vi "SMain.vi"() -> ()   [LabVIEW 2011] (continued)
0.283628\t0.245762\t0.211217\t0.212405\t0.226173\t0.234537\t0.236943\t0.231864\t0.218697\t0.203239\t0.212648\t0.219975\t0.225754\t0.228965\t0.229842\t0.227372\t0.235008\t0.246799\t0.255143\t0.261054\t0.264959\t0.267617\t0.269243\t0.269330\t0.267908\t0.264189\t0.257117\t0.251459\t0.263708\t0.269155\t0.266275\t0.292834\t0.323832\t0.346673\t0.359823\t0.362859\t0.356143\t0.340301\t0.316382\t0.287617\t0.273147\t0.255370\t0.232779\t0.205366\t0.184259\t0.170019\t0.153921\t0.138670\t0.147883\t0.157027\t0.165968\t0.178336\t0.204158\t0.226001\t0.243359\t0.256761\t0.265807\t0.270629\t0.271087\t0.271595\t0.274347\t0.273205\t0.284365\t0.290284\t0.291349\t0.282591\t0.268256\t0.253620\t0.246165\t0.249064\t0.246551\t0.238815\t0.226554\t0.210821\t0.192072\t0.170652\t0.155599\t0.155342\t0.161398\t0.165827\t0.167815\t0.166899\t0.173033\t0.183751\t0.192188\t0.212259\t0.241683\t0.269258\t0.293587\t0.314870\t0.333907\t0.351562\t0.368177\t0.383535\t0.397109\t0.407462\t0.412280\t0.409681\t0.419271\t0.438212\t0.456536\t0.460520\t0.453373\t0.437822\t0.419330\t0.400059\t0.375598\t0.345922\t0.315517\t0.294393\t0.276275\t0.256682\t0.235989\t0.212984\t0.221098\t0.231416\t0.236020\t0.246406\t0.268197\t0.283488\t0.291798\t0.294021\t0.290269\t0.280164\t0.264732\t0.299218\t0.335759\t0.373895\t0.412717\t0.447558\t0.468282\t0.461593\t0.427812\t0.447950\t0.482415\t0.501348\t0.510509\t0.512644\t0.508751\t0.498815\t0.483536\t0.485993\t0.477612\t0.457996\t0.425809\t0.384493\t0.344197\t0.326015\t0.302418\t0.272693\t0.237314\t0.216368\t0.210999\t0.199478\t0.207422\t0.232209\t0.251430\t0.266692\t0.284547\t0.301564\t0.329963\t0.366754\t0.402163\t0.427979\t0.426160\t0.475391\t0.545419\t0.537304\t0.479878\t0.459344\t0.451837\t0.454875\t0.465103\t0.478472\t0.489788\t0.494041\t0.487578\t0.468860\t0.438519\t0.399262\t0.353683\t0.305159\t0.285243\t0.282794\t0.274771\t0.260306\t0.239832\t0.212870\t0.186954\t0.181018\t0.172682\t0.162741\t0.164205\t0.181691\t0.197406\t0.217042\t0.241977\t0.265612\t0.291513\t0.357547\t0.416207\t0.466336\t0.534557\t0.484360\t0.426967\t0.399242\t0.390179\t0.380132\t0.376954\t0.366830\t0.349703\t0.326406\t0.298792\t0.270192\t0.250152\t0.237509\t0.223353\t0.207727\t0.191599\t0.198789\t0.207616\t0.242361\t0.266834\t0.281833\t0.287549\t0.284975\t0.274905\t0.258380\t0.235371\t0.206881\t0.203974\t0.229886\t0.255407\t0.280368\t0.310090\t0.346393\t0.328419\t0.547614\t0.529029\t0.416521\t0.384530\t0.347957\t0.317457\t0.289868\t0.261307\t0.245565\t0.261859\t0.294259\t0.327642\t0.358488\t0.365440\t0.348072\t0.309690\t0.255227\t0.240856\t0.244745\t0.245644\t0.243448\t0.267308\t0.282974\t0.288154\t0.284990\t0.275718\t0.261981\t0.265585\t0.277745\t0.291323\t0.306635\t0.334255\t0.362487\t0.382155\t0.353107\t0.253723\t0.328487\t0.577657\t0.533197\t0.444535\t0.396380\t0.364336\t0.339954\t0.349876\t0.362823\t0.384932\t0.406211\t0.413308\t0.403604\t0.377026\t0.337623\t0.289783\t0.272802\t0.257998\t0.243067\t0.227691\t0.221062\t0.216984\t0.213519\t0.223928\t0.234176\t0.242151\t0.248691\t0.253760\t0.258533\t0.263086\t0.267987\t0.273321\t0.287187\t0.311427\t0.320659\t0.286503\t0.237761\t0.343422\t0.397936\t0.389088\t0.372420\t0.361320\t0.354887\t0.367300\t0.377100\t0.380880\t0.381876\t0.383263\t0.385396\t0.387321\t0.387314\t0.384670\t0.378768\t0.373171\t0.363294\t0.348426\t0.328810\t0.313661\t0.308140\t0.297820\t0.282779\t0.263614\t0.241021\t0.215664\t0.214650\t0.218524\t0.229368\t0.253303\t0.273400\t0.292726\t0.295180\t0.280740\t0.235075\t0.247165\t0.271864\t0.272601\t0.263658\t0.258491\t0.263036\t0.264623\t0.267156\t0.272119\t0.286296\t0.307948\t0.326343\t0.339551\t0.347695\t0.356165\t0.365090\t0.365929\t0.359185\t0.345101\t0.324021\t0.297159\t0.290971\t0.280471\t0.265929\t0.248134\t0.226787\t0.219501\t0.263268\t0.311418\t0.359460\t0.406412\t0.446072\t0.458457\t0.418051\t0.344402\t0.280814\t0.230547\t0.208763\t0.198393\t0.193984\t0.208428\t0.213708\t0.210549\t0.232831\t0.253343\t0.270174\t0.282384\t0.288428\t0.289253\t0.284449\t0.278158\t0.286162\t0.291709\t0.290978\t0.284685\t0.271977\t0.261930\t0.261843\t0.260557\t0.272878\t0.283097\t0.291201\t0.297702\t0.324738\t0.371822\t0.417347\t0.457160\t0.481983\t0.480434\t0.450945\t0.404940\t0.353302\t0.301366\t0.250340\t0.199463\t0.149905\t0.148044\t0.164917\t0.193805\t0.216060\t0.231730\t0.241425\t0.245345\t0.251396\t0.261354\t0.272109\t0.277008\t0.273982\t0.263905\t0.248095\t0.229016\t0.209334\t0.206918\t0.200256\t0.189194\t0.178563\t0.201006\t0.223512\t0.256966\t0.308178\t0.367285\t0.414461\t0.444076\t0.452547\t0.440556\t0.413079\t0.375352\t0.330473\t0.279915\t0.224559\t0.238179\t0.268251\t0.289701\t0.303694\t0.311106\t0.323498\t0.342296\t0.355783\t0.363059\t0.364734\t0.372386\t0.382440\t0.387105\t0.386380\t0.380014\t0.367984\t0.354404\t0.334320\t0.305024\t0.270724\t0.253479\t0.229524\t0.240661\t0.278172\t0.303423\t0.309321\t0.327805\t0.352880\t0.365338\t0.363062\t0.345545\t0.341657\t0.327248\t0.302778\t0.298982\t0.305407\t0.328732\t0.351562\t0.367323\t0.377527\t0.381915\t0.380700\t0.389886\t0.411792\t0.429718\t0.443070\t0.452189\t0.462028\t0.484533\t0.500970\t0.511585\t0.516472\t0.514869\t0.506859\t0.490042\t0.463092\t0.423348\t0.387697\t0.420283\t0.472795\t0.503287\t0.496605\t0.466110\t0.425165\t0.380234\t0.405919\t0.428246\t0.440520\t0.443040\t0.436016\t0.445391\t0.459226\t0.464376\t0.461519\t0.463782\t0.470042\t0.477734\t0.478099\t0.471522\t0.457734\t0.436599\t0.407482\t0.409522\t0.412435\t0.410855\t0.409858\t0.441504\t0.471085\t0.494884\t0.511916\t0.520217\t0.515811\t0.493593\t0.461473\t0.504275\t0.528907\t0.545940\t0.525848\t0.492871\t0.457356\t0.421811\t0.390188\t0.421623\t0.444622\t0.459503\t0.466499\t0.465399\t0.485211\t0.508342\t0.522057\t0.529166\t0.532661\t0.528202\t0.516283\t0.497511\t0.477618\t0.455396\t0.429103\t0.409839\t0.422814\t0.433580\t0.441468\t0.445063\t0.441505\t0.425413\t0.423568\t0.444595\t0.469483\t0.470244\t0.504422\t0.538810\t0.510307\t0.481224\t0.464360\t0.435482\t0.401512\t0.365738\t0.351663\t0.347792\t0.374340\t0.394838\t0.410657\t0.422636\t0.428568\t0.455461\t0.473935\t0.486501\t0.489080\t0.483415\t0.472741\t0.455953\t0.435971\t0.414313\t0.388283\t0.356923\t0.319829\t0.303499\t0.304199\t0.299926\t0.317529\t0.357519\t0.387193\t0.400232\t0.416388\t0.500520\t0.560550\t0.540864\t0.459527\t0.362457\t0.272386\t0.273714\t0.283399\t0.288175\t0.289507\t0.287334\t0.329713\t0.382820\t0.427099\t0.462841\t0.490597\t0.510557\t0.523304\t0.529592\t0.529644\t0.524214\t0.513381\t0.497513\t0.476542\t0.450552\t0.419506\t0.383069\t0.340788\t0.314518\t0.301862\t0.285418\t0.263462\t0.286474\t0.325141\t0.370395\t0.457672\t0.528673\t0.581745\t0.630440\t0.558222\t0.459605\t0.359034\t0.256043\t0.186353\t0.196527\t0.223114\t0.287556\t0.343482\t0.392027\t0.433151\t0.466912\t0.493138\t0.511885\t0.522375\t0.525247\t0.522661\t0.516170\t0.503255\t0.483593\t0.457521\t0.424744\t0.385247\t0.337875\t0.281986\t0.222332\t0.196464\t0.168315\t0.199827\t0.297894\t0.393688\t0.485674\t0.566418\t0.602390\t0.561914\t0.536383\t0.468234\t0.383735\t0.290171\t0.203294\t0.178384\t0.210509\t0.252834\t0.291136\t0.351988\t0.406299\t0.454014\t0.493145\t0.522706\t0.543349\t0.556171\t0.560777\t0.558044\t0.548310\t0.531609\t0.507914\t0.477059\t0.438688\t0.391758\t0.335510\t0.268462\t0.189937\t0.194836\t0.216142\t0.289303\t0.380077\t0.463169\t0.533036\t0.576586\t0.575110\t0.565734\t0.519516\t0.453580\t0.377901\t0.295142\t0.217327\t0.224530\t0.241548\t0.258810\t0.298433\t0.340211\t0.392148\t0.436929\t0.471555\t0.496820\t0.513586\t0.521902\t0.522678\t0.516093\t0.501947\t0.480688\t0.452230\t0.415769\t0.370593\t0.315865\t0.250062\t0.208029\t0.202220\t0.273491\t0.343790\t0.412406\t0.478453\t0.523029\t0.531626\t0.504386\t0.469927\t0.427337\t0.366285\t0.293579\t0.246633\t0.199839\t0.193240\t0.229121\t0.278636\t0.321381\t0.363778\t0.397804\t0.424215\t0.451528\t0.473408\t0.486991\t0.492257\t0.489773\t0.479697\t0.462200\t0.436921\t0.403425\t0.360622\t0.307463\t0.243094\t0.184691\t0.209702\t0.251723\t0.325476\t0.400921\t0.470003\t0.530259\t0.571112\t0.573487\t0.534825\t0.475632\t0.409566\t0.336649\t0.257237\t0.197933\t0.209001\t0.214909\t0.216695\t0.256190\t0.324325\t0.381754\t0.429322\t0.467371\t0.495988\t0.515274\t0.525368\t0.526234\t0.520614\t0.508597\t0.488112\t0.458790\t0.419525\t0.369464\t0.307098\t0.238203\t0.242228\t0.265368\t0.300661\t0.344032\t0.410603\t0.479673\t0.534824\t0.571454\t0.602830\t0.596127\t0.555797\t0.497616\t0.429305\t0.369440\t0.362815\t0.348104\t0.334447\t0.344405\t0.359822\t0.388094\t0.413667\t0.433616\t0.447982\t0.477571\t0.510696\t0.535494\t0.556379\t0.568836\t0.572953\t0.567774\t0.552167\t0.524242\t0.482388\t0.424709\t0.349650\t0.281009\t0.293141\t0.324182\t0.376542\t0.428911\t0.469606\t0.504124\t0.525933\t0.566340\t0.582894\t0.565709\t0.526939\t0.476831\t0.419808\t0.356430\t0.375996\t0.389325\t0.394846\t0.438324\t0.471657\t0.494369\t0.508208\t0.514595\t0.514534\t0.508563\t0.503983\t0.493846\t0.476518\t0.482266\t0.493088\t0.498311\t0.498172\t0.491813\t0.477354\t0.450623\t0.419694\t0.420469\t0.406702\t0.449165\t0.484928\t0.537284\t0.568439\t0.564549\t0.526264\t0.513586\t0.483592\t0.436907\t0.408022\t0.371531\t0.330444\t0.285175\t0.269758\t0.314643\t0.382234\t0.437532\t0.481159\t0.513885\t0.536591\t0.549875\t0.554426\t0.550873\t0.539049\t0.519095\t0.490678\t0.452702\t0.404557\t0.345193\t0.279027\t0.208926\t0.188780\t0.204172\t0.285686\t0.356868\t0.417221\t0.464399\t0.495873\t0.549856\t0.578829\t0.568718\t0.527730\t0.470061\t0.402511\t0.344606\t0.281995\t0.231645\t0.219810\t0.208184\t0.213811\t0.261394\t0.306970\t0.358330\t0.405302\t0.442232\t0.469227\t0.487278\t0.496263\t0.496249\t0.487766\t0.470779\t0.445359\t0.411061\t0.367520\t0.351049\t0.349671\t0.370138\t0.381358\t0.418282\t0.450278\t0.473128\t0.483470\t0.478606\t0.475260\t0.479347\t0.483894\t0.466262\t0.439077\t0.399049\t0.350279\t0.356069\t0.385474\t0.407836\t0.429011\t0.450986\t0.462125\t0.477665\t0.489562\t0.492232\t0.487732\t0.476318\t0.458745\t0.451629\t0.447323\t0.433005\t0.408337\t0.372742\t0.326121\t0.302166\t0.275420\t0.283692\t0.335462\t0.375904\t0.405174\t0.444641\t0.477024\t0.509659\t0.527287\t0.528099\t0.512153\t0.480891\t0.446450\t0.405819\t0.370155\t0.325004\t0.317091\t0.329503\t0.333984\t0.352630\t0.380560\t0.396845\t0.402644\t0.452431\t0.496921\t0.531289\t0.555002\t0.566928\t0.565978\t0.551443\t0.522857\t0.480125\t0.432074\t0.412920\t0.388243\t0.366711\t0.391066\t0.441269\t0.496425\t0.545376\t0.582830\t0.604194\t0.643929\t0.648619\t0.615624\t0.573572\t0.524660\t0.470410\t0.409949\t0.341730\t0.333469\t0.320281\t0.338808\t0.377347\t0.450598\t0.521221\t0.577536\t0.612709\t0.620570\t0.607012\t0.585988\t0.569740\t0.596697\t0.615589\t0.625074\t0.624250\t0.611104\t0.583775\t0.541273\t0.482818\t0.425523\t0.402684\t0.375029\t0.405172\t0.472541\t0.534364\t0.589427\t0.631385\t0.644305\t0.696630\t0.726898\t0.670819\t0.611493\t0.553228\t0.496096\t0.435503\t0.369117\t0.326541\t0.322722\t0.365619\t0.455135\t0.537005\t0.604795\t0.650551\t0.659845\t0.634266\t0.589969\t0.544563\t0.543038\t0.566033\t0.579752\t0.583902\t0.577357\t0.559192\t0.528044\t0.482959\t0.473916\t0.467569\t0.466798\t0.516529\t0.565986\t0.625401\t0.682654\t0.738689\t0.768686\t0.723737\t0.664643\t0.668513\t0.648942\t0.606669\t0.548689\t0.478729\t0.416653\t0.393396\t0.405301\t0.463639\t0.502262\t0.521920\t0.541442\t0.615764\t0.679112\t0.717213\t0.697073\t0.643352\t0.580514\t0.538723\t0.543622\t0.542648\t0.534707\t0.528432\t0.530172\t0.518495\t0.496118\t0.464957\t0.480032\t0.524973\t0.563766\t0.586576\t0.591948\t0.596186\t0.626183\t0.644569\t0.644771\t0.622742\t0.582121\t0.547187\t0.503721\t0.452912\t0.395361\t0.399924\t0.416756\t0.427056\t0.462622\t0.483459\t0.485498\t0.521835\t0.571251\t0.601303\t0.599222\t0.563134\t0.504997\t0.456226\t0.472383\t0.494940\t0.539548\t0.568317\t0.572056\t0.553244\t0.519514\t0.476010\t0.453420\t0.489455\t0.519267\t0.531145\t0.525721\t0.505641\t0.474430\t0.460246\t0.438145\t0.428223\t0.421217\t0.407486\t0.388276\t0.386569\t0.410844\t0.429081\t0.440012\t0.441823\t0.432587\t0.414508\t0.407526\t0.437521\t0.473799\t0.498390\t0.506650\t0.494787\t0.461595\t0.409666\t0.341647\t0.373382\t0.442667\t0.508897\t0.575264\t0.642191\t0.663048\t0.598512\t0.521720\t0.441507\t0.397262\t0.401391\t0.396607\t0.383886\t0.364256\t0.361834\t0.382014\t0.393293\t0.396638\t0.408296\t0.435949\t0.453622\t0.461256\t0.458790\t0.446197\t0.423763\t0.391947\t0.351378\t0.325228\t0.323591\t0.332213\t0.331860\t0.321746\t0.300427\t0.279036\t0.285285\t0.289284\t0.348673\t0.402814\t0.454151\t0.505876\t0.560490\t0.619477\t0.648206\t0.581997\t0.490788\t0.392154\t0.327889\t0.294591\t0.241517\t0.183914\t0.244860\t0.340821\t0.417223\t0.476339\t0.519139\t0.545132\t0.553091\t0.543649\t0.520182\t0.486447\t0.445854\t0.400016\t0.348705\t0.317378\t0.296637\t0.270253\t0.253022\t0.256487\t0.281300\t0.329629\t0.373549\t0.405454\t0.423140\t0.426175\t0.467618\t0.500448\t0.524604\t0.578041\t0.648927\t0.768815\t0.611204\t0.499742\t0.385965\t0.410939\t0.460363\t0.476248\t0.427084\t0.382432\t0.431486\t0.510854\t0.571616\t0.609242\t0.616236\t0.597115\t0.564786\t0.526904\t0.485527\t0.441142\t0.393066\t0.340714\t0.312720\t0.283130\t0.274617\t0.317943\t0.365852\t0.415609\t0.463028\t0.501034\t0.520392\t0.514781\t0.487333\t0.470956\t0.477926\t0.469899\t0.455372\t0.496003\t0.556269\t0.638059\t0.657762\t0.523704\t0.437292\t0.379563\t0.477568\t0.547877\t0.547803\t0.554779\t0.608169\t0.629652\t0.608660\t0.569138\t0.530166\t0.495117\t0.458057\t0.418250\t0.374444\t0.326581\t0.304486\t0.309894\t0.325427\t0.338649\t0.352519\t0.382272\t0.437265\t0.511846\t0.575378\t0.602752\t0.576762\t0.527943\t0.476567\t0.426531\t0.377757\t0.402903\t0.426040\t0.446072\t0.460736\t0.464301\t0.459479\t0.466591\t0.455818\t0.520123\t0.576969\t0.642519\t0.698880\t0.708516\t0.671105\t0.628935\t0.586976\t0.543354\t0.496169\t0.443443\t0.383189\t0.337040\t0.340225\t0.342015\t0.383194\t0.434352\t0.481352\t0.516829\t0.541320\t0.535486\t0.534695\t0.603454\t0.636773\t0.614150\t0.567494\t0.517425\t0.467899\t0.440850\t0.440765\t0.432974\t0.415287\t0.400566\t0.410859\t0.468748\t0.527456\t0.583222\t0.623550\t0.654776\t0.664060\t0.647281\t0.612904\t0.568995\t0.522635\t0.481019\t0.433459\t0.378471\t0.315361\t0.243094\t0.248332\t0.307193\t0.377542\t0.451180\t0.530402\t0.620129\t0.720620\t0.647989\t0.563797\t0.513044\t0.540331\t0.547544\t0.534369\t0.506213\t0.468360\t0.472190\t0.474080\t0.467050\t0.459976\t0.471495\t0.506108\t0.561024\t0.608718\t0.643715\t0.656606\t0.643965\t0.615051\t0.577670\t0.534509\r\n*0.000000\t0.001250\t0.002501\t0.003751\t0.005001\t0.006252\t0.007502\t0.008752\t0.010003\t0.011253\t0.012503\t0.013753\t0.015004\t0.016254\t0.017504\t0.018755\t0.020005\t0.021255\t0.022506\t0.023756\t0.025006\t0.026257\t0.027507\t0.028757\t0.030008\t0.031258\t0.032508\t0.033758\t0.035009\t0.036259\t0.037509\t0.038760\t0.040010\t0.041260\t0.042511\t0.043761\t0.045011\t0.046262\t0.047512\t0.048762\t0.050013\t0.051263\t0.052513\t0.053763\t0.055014\t0.056264\t0.057514\t0.058765\t0.060015\t0.061265\t0.062516\t0.063766\t0.065016\t0.066267\t0.067517\t0.068767\t0.070018\t0.071268\t0.072518\t0.073768\t0.075019\t0.076269\t0.077519\t0.078770\t0.080020\t0.081270\t0.082521\t0.083771\t0.085021\t0.086272\t0.087522\t0.088772\t0.090023\t0.091273\t0.092523\t0.093773\t0.095024\t0.096274\t0.097524\t0.098775\t0.100025\t0.101275\t0.102526\t0.103776\t0.105026\t0.106277\t0.107527\t0.108777\t0.110028\t0.111278\t0.112528\t0.113778\t0.115029\t0.116279\t0.117529\t0.118780\t0.120030\t0.121280\t0.122531\t0.123781\t0.125031\t0.126282\t0.127532\t0.128782\t0.130033\t0.131283\t0.132533\t0.133783\t0.135034\t0.136284\t0.137534\t0.138785\t0.140035\t0.141285\t0.142536\t0.143786\t0.145036\t0.146287\t0.147537\t0.148787\t0.150038\t0.151288\t0.152538\t0.153788\t0.155039\t0.156289\t0.157539\t0.158790\t0.160040\t0.161290\t0.162541\t0.163791\t0.165041\t0.166292\t0.167542\t0.168792\t0.170043\t0.171293\t0.172543\t0.173793\t0.175044\t0.176294\t0.177544\t0.178795\t0.180045\t0.181295\t0.182546\t0.183796\t0.185046\t0.186297\t0.187547\t0.188797\t0.190048\t0.191298\t0.192548\t0.193798\t0.195049\t0.196299\t0.197549\t0.198800\t0.200050\t0.201300\t0.202551\t0.203801\t0.205051\t0.206302\t0.207552\t0.208802\t0.210053\t0.211303\t0.212553\t0.213803\t0.215054\t0.216304\t0.217554\t0.218805\t0.220055\t0.221305\t0.222556\t0.223806\t0.225056\t0.226307\t0.227557\t0.228807\t0.230058\t0.231308\t0.232558\t0.233808\t0.235059\t0.236309\t0.237559\t0.238810\t0.240060\t0.241310\t0.242561\t0.243811\t0.245061\t0.246312\t0.247562\t0.248812\t0.250063\t0.251313\t0.252563\t0.253813\t0.255064\t0.256314\t0.257564\t0.258815\t0.260065\t0.261315\t0.262566\t0.263816\t0.265066\t0.266317\t0.267567\t0.268817\t0.270068\t0.271318\t0.272568\t0.273818\t0.275069\t0.276319\t0.277569\t0.278820\t0.280070\t0.281320\t0.282571\t0.283821\t0.285071\t0.286322\t0.287572\t0.288822\t0.290073\t0.291323\t0.292573\t0.293823\t0.295074\t0.296324\t0.297574\t0.298825\t0.300075\t0.301325\t0.302576\t0.303826\t0.305076\t0.306327\t0.307577\t0.308827\t0.310078\t0.311328\t0.312578\t0.313828\t0.315079\t0.316329\t0.317579\t0.318830\t0.320080\t0.321330\t0.322581\t0.323831\t0.325081\t0.326332\t0.327582\t0.328832\t0.330083\t0.331333\t0.332583\t0.333833\t0.335084\t0.336334\t0.337584\t0.338835\t0.340085\t0.341335\t0.342586\t0.343836\t0.345086\t0.346337\t0.347587\t0.348837\t0.350088\t0.351338\t0.352588\t0.353838\t0.355089\t0.356339\t0.357589\t0.358840\t0.360090\t0.361340\t0.362591\t0.363841\t0.365091\t0.366342\t0.367592\t0.368842\t0.370093\t0.371343\t0.372593\t0.373843\t0.375094\t0.376344\t0.377594\t0.378845\t0.380095\t0.381345\t0.382596\t0.383846\t0.385096\t0.386347\t0.387597\t0.388847\t0.390098\t0.391348\t0.392598\t0.393848\t0.395099\t0.396349\t0.397599\t0.398850\t0.400100\t0.401350\t0.402601\t0.403851\t0.405101\t0.406352\t0.407602\t0.408852\t0.410103\t0.411353\t0.412603\t0.413853\t0.415104\t0.416354\t0.417604\t0.418855\t0.420105\t0.421355\t0.422606\t0.423856\t0.425106\t0.426357\t0.427607\t0.428857\t0.430108\t0.431358\t0.432608\t0.433858\t0.435109\t0.436359\t0.437609\t0.438860\t0.440110\t0.441360\t0.442611\t0.443861\t0.445111\t0.446362\t0.447612\t0.448862\t0.450113\t0.451363\t0.452613\t0.453863\t0.455114\t0.456364\t0.457614\t0.458865\t0.460115\t0.461365\t0.462616\t0.463866\t0.465116\t0.466367\t0.467617\t0.468867\t0.470118\t0.471368\t0.472618\t0.473868\t0.475119\t0.476369\t0.477619\t0.478870\t0.480120\t0.481370\t0.482621\t0.483871\t0.485121\t0.486372\t0.487622\t0.488872\t0.490123\t0.491373\t0.492623\t0.493873\t0.495124\t0.496374\t0.497624\t0.498875\t0.500125\t0.501375\t0.502626\t0.503876\t0.505126\t0.506377\t0.507627\t0.508877\t0.510128\t0.511378\t0.512628\t0.513878\t0.515129\t0.516379\t0.517629\t0.518880\t0.520130\t0.521380\t0.522631\t0.523881\t0.525131\t0.526382\t0.527632\t0.528882\t0.530133\t0.531383\t0.532633\t0.533883\t0.535134\t0.536384\t0.537634\t0.538885\t0.540135\t0.541385\t0.542636\t0.543886\t0.545136\t0.546387\t0.547637\t0.548887\t0.550138\t0.551388\t0.552638\t0.553888\t0.555139\t0.556389\t0.557639\t0.558890\t0.560140\t0.561390\t0.562641\t0.563891\t0.565141\t0.566392\t0.567642\t0.568892\t0.570143\t0.571393\t0.572643\t0.573893\t0.575144\t0.576394\t0.577644\t0.578895\t0.580145\t0.581395\t0.582646\t0.583896\t0.585146\t0.586397\t0.587647\t0.588897\t0.590148\t0.591398\t0.592648\t0.593898\t0.595149\t0.596399\t0.597649\t0.598900\t0.600150\t0.601400\t0.602651\t0.603901\t0.605151\t0.606402\t0.607652\t0.608902\t0.610153\t0.611403\t0.612653\t0.613903\t0.615154\t0.616404\t0.617654\t0.618905\t0.620155\t0.621405\t0.622656\t0.623906\t0.625156\t0.626407\t0.627657\t0.628907\t0.630158\t0.631408\t0.632658\t0.633908\t0.635159\t0.636409\t0.637659\t0.638910\t0.640160\t0.641410\t0.642661\t0.643911\t0.645161\t0.646412\t0.647662\t0.648912\t0.650163\t0.651413\t0.652663\t0.653913\t0.655164\t0.656414\t0.657664\t0.658915\t0.660165\t0.661415\t0.662666\t0.663916\t0.665166\t0.666417\t0.667667\t0.668917\t0.670168\t0.671418\t0.672668\t0.673918\t0.675169\t0.676419\t0.677669\t0.678920\t0.680170\t0.681420\t0.682671\t0.683921\t0.685171\t0.686422\t0.687672\t0.688922\t0.690173\t0.691423\t0.692673\t0.693923\t0.695174\t0.696424\t0.697674\t0.698925\t0.700175\t0.701425\t0.702676\t0.703926\t0.705176\t0.706427\t0.707677\t0.708927\t0.710178\t0.711428\t0.712678\t0.713928\t0.715179\t0.716429\t0.717679\t0.718930\t0.720180\t0.721430\t0.722681\t0.723931\t0.725181\t0.726432\t0.727682\t0.728932\t0.730183\t0.731433\t0.732683\t0.733933\t0.735184\t0.736434\t0.737684\t0.738935\t0.740185\t0.741435\t0.742686\t0.743936\t0.745186\t0.746437\t0.747687\t0.748937\t0.750188\t0.751438\t0.752688\t0.753938\t0.755189\t0.756439\t0.757689\t0.758940\t0.760190\t0.761440\t0.762691\t0.763941\t0.765191\t0.766442\t0.767692\t0.768942\t0.770193\t0.771443\t0.772693\t0.773943\t0.775194\t0.776444\t0.777694\t0.778945\t0.780195\t0.781445\t0.782696\t0.783946\t0.785196\t0.786447\t0.787697\t0.788947\t0.790198\t0.791448\t0.792698\t0.793948\t0.795199\t0.796449\t0.797699\t0.798950\t0.800200\t0.801450\t0.802701\t0.803951\t0.805201\t0.806452\t0.807702\t0.808952\t0.810203\t0.811453\t0.812703\t0.813953\t0.815204\t0.816454\t0.817704\t0.818955\t0.820205\t0.821455\t0.822706\t0.823956\t0.825206\t0.826457\t0.827707\t0.828957\t0.830208\t0.831458\t0.832708\t0.833958\t0.835209\t0.836459\t0.837709\t0.838960\t0.840210\t0.841460\t0.842711\t0.843961\t0.845211\t0.846462\t0.847712\t0.848962\t0.850213\t0.851463\t0.852713\t0.853963\t0.855214\t0.856464\t0.857714\t0.858965\t0.860215\t0.861465\t0.862716\t0.863966\t0.865216\t0.866467\t0.867717\t0.868967\t0.870218\t0.871468\t0.872718\t0.873968\t0.875219\t0.876469\t0.877719\t0.878970\t0.880220\t0.881470\t0.882721\t0.883971\t0.885221\t0.886472\t0.887722\t0.888972\t0.890223\t0.891473\t0.892723\t0.893973\t0.895224\t0.896474\t0.897724\t0.898975\t0.900225\t0.901475\t0.902726\t0.903976\t0.905226\t0.906477\t0.907727\t0.908977\t0.910228\t0.911478\t0.912728\t0.913978\t0.915229\t0.916479\t0.917729\t0.918980\t0.920230\t0.921480\t0.922731\t0.923981\t0.925231\t0.926482\t0.927732\t0.928982\t0.930233\t0.931483\t0.932733\t0.933983\t0.935234\t0.936484\t0.937734\t0.938985\t0.940235\t0.941485\t0.942736\t0.943986\t0.945236\t0.946487\t0.947737\t0.948987\t0.950238\t0.951488\t0.952738\t0.953988\t0.955239\t0.956489\t0.957739\t0.958990\t0.960240\t0.961490\t0.962741\t0.963991\t0.965241\t0.966492\t0.967742\t0.968992\t0.970243\t0.971493\t0.972743\t0.973993\t0.975244\t0.976494\t0.977744\t0.978995\t0.980245\t0.981495\t0.982746\t0.983996\t0.985246\t0.986497\t0.987747\t0.988997\t0.990248\t0.991498\t0.992748\t0.993998\t0.995249\t0.996499\t0.997749\t0.999000\t1.000250\t1.001500\t1.002751\t1.004001\t1.005251\t1.006502\t1.007752\t1.009002\t1.010253\t1.011503\t1.012753\t1.014004\t1.015254\t1.016504\t1.017754\t1.019005\t1.020255\t1.021505\t1.022756\t1.024006\t1.025256\t1.026507\t1.027757\t1.029007\t1.030258\t1.031508\t1.032758\t1.034009\t1.035259\t1.036509\t1.037759\t1.039010\t1.040260\t1.041510\t1.042761\t1.044011\t1.045261\t1.046512\t1.047762\t1.049012\t1.050263\t1.051513\t1.052763\t1.054014\t1.055264\t1.056514\t1.057764\t1.059015\t1.060265\t1.061515\t1.062766\t1.064016\t1.065266\t1.066517\t1.067767\t1.069017\t1.070268\t1.071518\t1.072768\t1.074019\t1.075269\t1.076519\t1.077769\t1.079020\t1.080270\t1.081520\t1.082771\t1.084021\t1.085271\t1.086522\t1.087772\t1.089022\t1.090273\t1.091523\t1.092773\t1.094024\t1.095274\t1.096524\t1.097774\t1.099025\t1.100275\t1.101525\t1.102776\t1.104026\t1.105276\t1.106527\t1.107777\t1.109027\t1.110278\t1.111528\t1.112778\t1.114029\t1.115279\t1.116529\t1.117779\t1.119030\t1.120280\t1.121530\t1.122781\t1.124031\t1.125281\t1.126532\t1.127782\t1.129032\t1.130283\t1.131533\t1.132783\t1.134034\t1.135284\t1.136534\t1.137784\t1.139035\t1.140285\t1.141535\t1.142786\t1.144036\t1.145286\t1.146537\t1.147787\t1.149037\t1.150288\t1.151538\t1.152788\t1.154039\t1.155289\t1.156539\t1.157789\t1.159040\t1.160290\t1.161540\t1.162791\t1.164041\t1.165291\t1.166542\t1.167792\t1.169042\t1.170293\t1.171543\t1.172793\t1.174044\t1.175294\t1.176544\t1.177794\t1.179045\t1.180295\t1.181545\t1.182796\t1.184046\t1.185296\t1.186547\t1.187797\t1.189047\t1.190298\t1.191548\t1.192798\t1.194049\t1.195299\t1.196549\t1.197799\t1.199050\t1.200300\t1.201550\t1.202801\t1.204051\t1.205301\t1.206552\t1.207802\t1.209052\t1.210303\t1.211553\t1.212803\t1.214054\t1.215304\t1.216554\t1.217804\t1.219055\t1.220305\t1.221555\t1.222806\t1.224056\t1.225306\t1.226557\t1.227807\t1.229057\t1.230308\t1.231558\t1.232808\t1.234059\t1.235309\t1.236559\t1.237809\t1.239060\t1.240310\t1.241560\t1.242811\t1.244061\t1.245311\t1.246562\t1.247812\t1.249062\t1.250313\t1.251563\t1.252813\t1.254064\t1.255314\t1.256564\t1.257814\t1.259065\t1.260315\t1.261565\t1.262816\t1.264066\t1.265316\t1.266567\t1.267817\t1.269067\t1.270318\t1.271568\t1.272818\t1.274069\t1.275319\t1.276569\t1.277819\t1.279070\t1.280320\t1.281570\t1.282821\t1.284071\t1.285321\t1.286572\t1.287822\t1.289072\t1.290323\t1.291573\t1.292823\t1.294074\t1.295324\t1.296574\t1.297824\t1.299075\t1.300325\t1.301575\t1.302826\t1.304076\t1.305326\t1.306577\t1.307827\t1.309077\t1.310328\t1.311578\t1.312828\t1.314079\t1.315329\t1.316579\t1.317829\t1.319080\t1.320330\t1.321580\t1.322831\t1.324081\t1.325331\t1.326582\t1.327832\t1.329082\t1.330333\t1.331583\t1.332833\t1.334084\t1.335334\t1.336584\t1.337834\t1.339085\t1.340335\t1.341585\t1.342836\t1.344086\t1.345336\t1.346587\t1.347837\t1.349087\t1.350338\t1.351588\t1.352838\t1.354089\t1.355339\t1.356589\t1.357839\t1.359090\t1.360340\t1.361590\t1.362841\t1.364091\t1.365341\t1.366592\t1.367842\t1.369092\t1.370343\t1.371593\t1.372843\t1.374094\t1.375344\t1.376594\t1.377844\t1.379095\t1.380345\t1.381595\t1.382846\t1.384096\t1.385346\t1.386597\t1.387847\t1.389097\t1.390348\t1.391598\t1.392848\t1.394099\t1.395349\t1.396599\t1.397849\t1.399100\t1.400350\t1.401600\t1.402851\t1.404101\t1.405351\t1.406602\t1.407852\t1.409102\t1.410353\t1.411603\t1.412853\t1.414104\t1.415354\t1.416604\t1.417854\t1.419105\t1.420355\t1.421605\t1.422856\t1.424106\t1.425356\t1.426607\t1.427857\t1.429107\t1.430358\t1.431608\t1.432858\t1.434109\t1.435359\t1.436609\t1.437859\t1.439110\t1.440360\t1.441610\t1.442861\t1.444111\t1.445361\t1.446612\t1.447862\t1.449112\t1.450363\t1.451613\t1.452863\t1.454114\t1.455364\t1.456614\t1.457864\t1.459115\t1.460365\t1.461615\t1.462866\t1.464116\t1.465366\t1.466617\t1.467867\t1.469117\t1.470368\t1.471618\t1.472868\t1.474119\t1.475369\t1.476619\t1.477869\t1.479120\t1.480370\t1.481620\t1.482871\t1.484121\t1.485371\t1.486622\t1.487872\t1.489122\t1.490373\t1.491623\t1.492873\t1.494124\t1.495374\t1.496624\t1.497874\t1.499125\t1.500375\t1.501625\t1.502876\t1.504126\t1.505376\t1.506627\t1.507877\t1.509127\t1.510378\t1.511628\t1.512878\t1.514129\t1.515379\t1.516629\t1.517879\t1.519130\t1.520380\t1.521630\t1.522881\t1.524131\t1.525381\t1.526632\t1.527882\t1.529132\t1.530383\t1.531633\t1.532883\t1.534134\t1.535384\t1.536634\t1.537884\t1.539135\t1.540385\t1.541635\t1.542886\t1.544136\t1.545386\t1.546637\t1.547887\t1.549137\t1.550388\t1.551638\t1.552888\t1.554139\t1.555389\t1.556639\t1.557889\t1.559140\t1.560390\t1.561640\t1.562891\t1.564141\t1.565391\t1.566642\t1.567892\t1.569142\t1.570393\t1.571643\t1.572893\t1.574144\t1.575394\t1.576644\t1.577894\t1.579145\t1.580395\t1.581645\t1.582896\t1.584146\t1.585396\t1.586647\t1.587897\t1.589147\t1.590398\t1.591648\t1.592898\t1.594149\t1.595399\t1.596649\t1.597899\t1.599150\t1.600400\t1.601650\t1.602901\t1.604151\t1.605401\t1.606652\t1.607902\t1.609152\t1.610403\t1.611653\t1.612903\t1.614154\t1.615404\t1.616654\t1.617904\t1.619155\t1.620405\t1.621655\t1.622906\t1.624156\t1.625406\t1.626657\t1.627907\t1.629157\t1.630408\t1.631658\t1.632908\t1.634159\t1.635409\t1.636659\t1.637909\t1.639160\t1.640410\t1.641660\t1.642911\t1.644161\t1.645411\t1.646662\t1.647912\t1.649162\t1.650413\t1.651663\t1.652913\t1.654164\t1.655414\t1.656664\t1.657914\t1.659165\t1.660415\t1.661665\t1.662916\t1.664166\t1.665416\t1.666667\t1.667917\t1.669167\t1.670418\t1.671668\t1.672918\t1.674169\t1.675419\t1.676669\t1.677919\t1.679170\t1.680420\t1.681670\t1.682921\t1.684171\t1.685421\t1.686672\t1.687922\t1.689172\t1.690423\t1.691673\t1.692923\t1.694174\t1.695424\t1.696674\t1.697924\t1.699175\t1.700425\t1.701675\t1.702926\t1.704176\t1.705426\t1.706677\t1.707927\t1.709177\t1.710428\t1.711678\t1.712928\t1.714179\t1.715429\t1.716679\t1.717929\t1.719180\t1.720430\t1.721680\t1.722931\t1.724181\t1.725431\t1.726682\t1.727932\t1.729182\t1.730433\t1.731683\t1.732933\t1.734184\t1.735434\t1.736684\t1.737934\t1.739185\t1.740435\t1.741685\t1.742936\t1.744186\t1.745436\t1.746687\t1.747937\t1.749187\t1.750438\t1.751688\t1.752938\t1.754189\t1.755439\t1.756689\t1.757939\t1.759190\t1.760440\t1.761690\t1.762941\t1.764191\t1.765441\t1.766692\t1.767942\t1.769192\t1.770443\t1.771693\t1.772943\t1.774194\t1.775444\t1.776694\t1.777944\t1.779195\t1.780445\t1.781695\t1.782946\t1.784196\t1.785446\t1.786697\t1.787947\t1.789197\t1.790448\t1.791698\t1.792948\t1.794199\t1.795449\t1.796699\t1.797949\t1.799200\t1.800450\t1.801700\t1.802951\t1.804201\t1.805451\t1.806702\t1.807952\t1.809202\t1.810453\t1.811703\t1.812953\t1.814204\t1.815454\t1.816704\t1.817954\t1.819205\t1.820455\t1.821705\t1.822956\t1.824206\t1.825456\t1.826707\t1.827957\t1.829207\t1.830458\t1.831708\t1.832958\t1.834209\t1.835459\t1.836709\t1.837959\t1.839210\t1.840460\t1.841710\t1.842961\t1.844211\t1.845461\t1.846712\t1.847962\t1.849212\t1.850463\t1.851713\t1.852963\t1.854214\t1.855464\t1.856714\t1.857964\t1.859215\t1.860465\t1.861715\t1.862966\t1.864216\t1.865466\t1.866717\t1.867967\t1.869217\t1.870468\t1.871718\t1.872968\t1.874219\t1.875469\t1.876719\t1.877969\t1.879220\t1.880470\t1.881720\t1.882971\t1.884221\t1.885471\t1.886722\t1.887972\t1.889222\t1.890473\t1.891723\t1.892973\t1.894224\t1.895474\t1.896724\t1.897974\t1.899225\t1.900475\t1.901725\t1.902976\t1.904226\t1.905476\t1.906727\t1.907977\t1.909227\t1.910478\t1.911728\t1.912978\t1.914229\t1.915479\t1.916729\t1.917979\t1.919230\t1.920480\t1.921730\t1.922981\t1.924231\t1.925481\t1.926732\t1.927982\t1.929232\t1.930483\t1.931733\t1.932983\t1.934234\t1.935484\t1.936734\t1.937984\t1.939235\t1.940485\t1.941735\t1.942986\t1.944236\t1.945486\t1.946737\t1.947987\t1.949237\t1.950488\t1.951738\t1.952988\t1.954239\t1.955489\t1.956739\t1.957989\t1.959240\t1.960490\t1.961740\t1.962991\t1.964241\t1.965491\t1.966742\t1.967992\t1.969242\t1.970493\t1.971743\t1.972993\t1.974244\t1.975494\t1.976744\t1.977994\t1.979245\t1.980495\t1.981745\t1.982996\t1.984246\t1.985496\t1.986747\t1.987997\t1.989247\t1.990498\t1.991748\t1.992998\t1.994249\t1.995499\t1.996749\t1.997999\t1.999250\t2.000500\t2.001750\t2.003001\t2.004251\t2.005501\t2.006752\t2.008002\t2.009252\t2.010503\t2.011753\t2.013003\t2.014254\t2.015504\t2.016754\t2.018005\t2.019255\t2.020505\t2.021755\t2.023006\t2.024256\t2.025506\t2.026757\t2.028007\t2.029257\t2.030508\t2.031758\t2.033008\t2.034259\t2.035509\t2.036759\t2.038010\t2.039260\t2.040510\t2.041760\t2.043011\t2.044261\t2.045511\t2.046762\t2.048012\t2.049262\t2.050513\t2.051763\t2.053013\t2.054264\t2.055514\t2.056764\t2.058015\t2.059265\t2.060515\t2.061765\t2.063016\t2.064266\t2.065516\t2.066767\t2.068017\t2.069267\t2.070518\t2.071768\t2.073018\t2.074269\t2.075519\t2.076769\t2.078020\t2.079270\t2.080520\t2.081770\t2.083021\t2.084271\t2.085521\t2.086772\t2.088022\t2.089272\t2.090523\t2.091773\t2.093023\t2.094274\t2.095524\t2.096774\t2.098025\t2.099275\t2.100525\t2.101775\t2.103026\t2.104276\t2.105526\t2.106777\t2.108027\t2.109277\t2.110528\t2.111778\t2.113028\t2.114279\t2.115529\t2.116779\t2.118030\t2.119280\t2.120530\t2.121780\t2.123031\t2.124281\t2.125531\t2.126782\t2.128032\t2.129282\t2.130533\t2.131783\t2.133033\t2.134284\t2.135534\t2.136784\t2.138035\t2.139285\t2.140535\t2.141785\t2.143036\t2.144286\t2.145536\t2.146787\t2.148037\t2.149287\t2.150538\t2.151788\t2.153038\t2.154289\t2.155539\t2.156789\t2.158040\t2.159290\t2.160540\t2.161790\t2.163041\t2.164291\t2.165541\t2.166792\t2.168042\t2.169292\t2.170543\t2.171793\t2.173043\t2.174294\t2.175544\t2.176794\t2.178045\t2.179295\t2.180545\t2.181795\t2.183046\t2.184296\t2.185546\t2.186797\t2.188047\t2.189297\t2.190548\t2.191798\t2.193048\t2.194299\t2.195549\t2.196799\t2.198050\t2.199300\t2.200550\t2.201800\t2.203051\t2.204301\t2.205551\t2.206802\t2.208052\t2.209302\t2.210553\t2.211803\t2.213053\t2.214304\t2.215554\t2.216804\t2.218055\t2.219305\t2.220555\t2.221805\t2.223056\t2.224306\t2.225556\t2.226807\t2.228057\t2.229307\t2.230558\t2.231808\t2.233058\t2.234309\t2.235559\t2.236809\t2.238060\t2.239310\t2.240560\t2.241810\t2.243061\t2.244311\t2.245561\t2.246812\t2.248062\t2.249312\t2.250563\t2.251813\t2.253063\t2.254314\t2.255564\t2.256814\t2.258065\t2.259315\t2.260565\t2.261815\t2.263066\t2.264316\t2.265566\t2.266817\t2.268067\t2.269317\t2.270568\t2.271818\t2.273068\t2.274319\t2.275569\t2.276819\t2.278070\t2.279320\t2.280570\t2.281820\t2.283071\t2.284321\t2.285571\t2.286822\t2.288072\t2.289322\t2.290573\t2.291823\t2.293073\t2.294324\t2.295574\t2.296824\t2.298075\t2.299325\t2.300575\t2.301825\t2.303076\t2.304326\t2.305576\t2.306827\t2.308077\t2.309327\t2.310578\t2.311828\t2.313078\t2.314329\t2.315579\t2.316829\t2.318080\t2.319330\t2.320580\t2.321830\t2.323081\t2.324331\t2.325581\t2.326832\t2.328082\t2.329332\t2.330583\t2.331833\t2.333083\t2.334334\t2.335584\t2.336834\t2.338085\t2.339335\t2.340585\t2.341835\t2.343086\t2.344336\t2.345586\t2.346837\t2.348087\t2.349337\t2.350588\t2.351838\t2.353088\t2.354339\t2.355589\t2.356839\t2.358090\t2.359340\t2.360590\t2.361840\t2.363091\t2.364341\t2.365591\t2.366842\t2.368092\t2.369342\t2.370593\t2.371843\t2.373093\t2.374344\t2.375594\t2.376844\t2.378095\t2.379345\t2.380595\t2.381845\t2.383096\t2.384346\t2.385596\t2.386847\t2.388097\t2.389347\t2.390598\t2.391848\t2.393098\t2.394349\t2.395599\t2.396849\t2.398100\t2.399350\t2.400600\t2.401850\t2.403101\t2.404351\t2.405601\t2.406852\t2.408102\t2.409352\t2.410603\t2.411853\t2.413103\t2.414354\t2.415604\t2.416854\t2.418105\t2.419355\t2.420605\t2.421855\t2.423106\t2.424356\t2.425606\t2.426857\t2.428107\t2.429357\t2.430608\t2.431858\t2.433108\t2.434359\t2.435609\t2.436859\t2.438110\t2.439360\t2.440610\t2.441860\t2.443111\t2.444361\t2.445611\t2.446862\t2.448112\t2.449362\t2.450613\t2.451863\t2.453113\t2.454364\t2.455614\t2.456864\t2.458115\t2.459365\t2.460615\t2.461865\t2.463116\t2.464366\t2.465616\t2.466867\t2.468117\t2.469367\t2.470618\t2.471868\t2.473118\t2.474369\t2.475619\t2.476869\t2.478120\t2.479370\t2.480620\t2.481870\t2.483121\t2.484371\t2.485621\t2.486872\t2.488122\t2.489372\t2.490623\t2.491873\t2.493123\t2.494374\t2.495624\t2.496874\t2.498125\t2.499375\t2.500625\t2.501875\t2.503126\t2.504376\t2.505626\t2.506877\t2.508127\t2.509377\t2.510628\t2.511878\t2.513128\t2.514379\t2.515629\t2.516879\t2.518130\t2.519380\t2.520630\t2.521880\t2.523131\t2.524381\t2.525631\t2.526882\t2.528132\t2.529382\t2.530633\t2.531883\t2.533133\t2.534384\t2.535634\t2.536884\t2.538135\t2.539385\t2.540635\t2.541885\t2.543136\t2.544386\t2.545636\t2.546887\t2.548137\t2.549387\t2.550638\t2.551888\t2.553138\t2.554389\t2.555639\t2.556889\t2.558140\t2.559390\t2.560640\t2.561890\t2.563141\t2.564391\t2.565641\t2.566892\t2.568142\t2.569392\t2.570643\t2.571893\t2.573143\t2.574394\t2.575644\t2.576894\t2.578145\t2.579395\t2.580645\t2.581895\t2.583146\t2.584396\t2.585646\t2.586897\t2.588147\t2.589397\t2.590648\t2.591898\t2.593148\t2.594399\t2.595649\t2.596899\t2.598150\t2.599400\t2.600650\t2.601900\t2.603151\t2.604401\t2.605651\t2.606902\t2.608152\t2.609402\t2.610653\t2.611903\t2.613153\t2.614404\t2.615654\t2.616904\t2.618155\t2.619405\t2.620655\t2.621905\t2.623156\t2.624406\t2.625656\t2.626907\t2.628157\t2.629407\t2.630658\t2.631908\t2.633158\t2.634409\t2.635659\t2.636909\t2.638160\t2.639410\t2.640660\t2.641910\t2.643161\t2.644411\t2.645661\t2.646912\t2.648162\t2.649412\t2.650663\t2.651913\t2.653163\t2.654414\t2.655664\t2.656914\t2.658165\t2.659415\t2.660665\t2.661915\t2.663166\t2.664416\t2.665666\t2.666917\t2.668167\t2.669417\t2.670668\t2.671918\t2.673168\t2.674419\t2.675669\t2.676919\t2.678170\t2.679420\t2.680670\t2.681920\t2.683171\t2.684421\t2.685671\t2.686922\t2.688172\t2.689422\t2.690673\t2.691923\t2.693173\t2.694424\t2.695674\t2.696924\t2.698175\t2.699425\t2.700675\t2.701925\t2.703176\t2.704426\t2.705676\t2.706927\t2.708177\t2.709427\t2.710678\t2.711928\t2.713178\t2.714429\t2.715679\t2.716929\t2.718180\t2.719430\t2.720680\t2.721930\t2.723181\t2.724431\t2.725681\t2.726932\t2.728182\t2.729432\t2.730683\t2.731933\t2.733183\t2.734434\t2.735684\t2.736934\t2.738185\t2.739435\t2.740685\t2.741935\t2.743186\t2.744436\t2.745686\t2.746937\t2.748187\t2.749437\t2.750688\t2.751938\t2.753188\t2.754439\t2.755689\t2.756939\t2.758190\t2.759440\t2.760690\t2.761940\t2.763191\t2.764441\t2.765691\t2.766942\t2.768192\t2.769442\t2.770693\t2.771943\t2.773193\t2.774444\t2.775694\t2.776944\t2.778195\t2.779445\t2.780695\t2.781945\t2.783196\t2.784446\t2.785696\t2.786947\t2.788197\t2.789447\t2.790698\t2.791948\t2.793198\t2.794449\t2.795699\t2.796949\t2.798200\t2.799450\t2.800700\t2.801950\t2.803201\t2.804451\t2.805701\t2.806952\t2.808202\t2.809452\t2.810703\t2.811953\t2.813203\t2.814454\t2.815704\t2.816954\t2.818205\t2.819455\t2.820705\t2.821955\t2.823206\t2.824456\t2.825706\t2.826957\t2.828207\t2.829457\t2.830708\t2.831958\t2.833208\t2.834459\t2.835709\t2.836959\t2.838210\t2.839460\t2.840710\t2.841960\t2.843211\t2.844461\t2.845711\t2.846962\t2.848212\t2.849462\t2.850713\t2.851963\t2.853213\t2.854464\t2.855714\t2.856964\t2.858215\t2.859465\t2.860715\t2.861965\t2.863216\t2.864466\t2.865716\t2.866967\t2.868217\t2.869467\t2.870718\t2.871968\t2.873218\t2.874469\t2.875719\t2.876969\t2.878220\t2.879470\t2.880720\t2.881970\t2.883221\t2.884471\t2.885721\t2.886972\t2.888222\t2.889472\t2.890723\t2.891973\t2.893223\t2.894474\t2.895724\t2.896974\t2.898225\t2.899475\t2.900725\t2.901975\t2.903226\t2.904476\t2.905726\t2.906977\t2.908227\t2.909477\t2.910728\t2.911978\t2.913228\t2.914479\t2.915729\t2.916979\t2.918230\t2.919480\t2.920730\t2.921980\t2.923231\t2.924481\t2.925731\t2.926982\t2.928232\t2.929482\t2.930733\t2.931983\t2.933233\t2.934484\t2.935734\t2.936984\t2.938235\t2.939485\t2.940735\t2.941985\t2.943236\t2.944486\t2.945736\t2.946987\t2.948237\t2.949487\t2.950738\t2.951988\t2.953238\t2.954489\t2.955739\t2.956989\t2.958240\t2.959490\t2.960740\t2.961990\t2.963241\t2.964491\t2.965741\t2.966992\t2.968242\t2.969492\t2.970743\t2.971993\t2.973243\t2.974494\t2.975744\t2.976994\t2.978245\t2.979495\t2.980745\t2.981995\t2.983246\t2.984496\t2.985746\t2.986997\t2.988247\t2.989497\t2.990748\t2.991998\t2.993248\t2.994499\t2.995749\t2.996999\t2.998250\t2.999500\t3.000750\t3.002001\t3.003251\t3.004501\t3.005751\t3.007002\t3.008252\t3.009502\t3.010753\t3.012003\t3.013253\t3.014504\t3.015754\t3.017004\t3.018255\t3.019505\t3.020755\t3.022006\t3.023256\t3.024506\t3.025756\t3.027007\t3.028257\t3.029507\t3.030758\t3.032008\t3.033258\t3.034509\t3.035759\t3.037009\t3.038260\t3.039510\t3.040760\t3.042011\t3.043261\t3.044511\t3.045761\t3.047012\t3.048262\t3.049512\t3.050763\t3.052013\t3.053263\t3.054514\t3.055764\t3.057014\t3.058265\t3.059515\t3.060765\t3.062016\t3.063266\t3.064516\t3.065766\t3.067017\t3.068267\t3.069517\t3.070768\t3.072018\t3.073268\t3.074519\t3.075769\t3.077019\t3.078270\t3.079520\t3.080770\t3.082021\t3.083271\t3.084521\t3.085771\t3.087022\t3.088272\t3.089522\t3.090773\t3.092023\t3.093273\t3.094524\t3.095774\t3.097024\t3.098275\t3.099525\t3.100775\t3.102026\t3.103276\t3.104526\t3.105776\t3.107027\t3.108277\t3.109527\t3.110778\t3.112028\t3.113278\t3.114529\t3.115779\t3.117029\t3.118280\t3.119530\t3.120780\t3.122031\t3.123281\t3.124531\t3.125781\t3.127032\t3.128282\t3.129532\t3.130783\t3.132033\t3.133283\t3.134534\t3.135784\t3.137034\t3.138285\t3.139535\t3.140785\t3.142036\t3.143286\t3.144536\t3.145786\t3.147037\t3.148287\t3.149537\t3.150788\t3.152038\t3.153288\t3.154539\t3.155789\t3.157039\t3.158290\t3.159540\t3.160790\t3.162041\t3.163291\t3.164541\t3.165791\t3.167042\t3.168292\t3.169542\t3.170793\t3.172043\t3.173293\t3.174544\t3.175794\t3.177044\t3.178295\t3.179545\t3.180795\t3.182046\t3.183296\t3.184546\t3.185796\t3.187047\t3.188297\t3.189547\t3.190798\t3.192048\t3.193298\t3.194549\t3.195799